vi "run.vi"(8 "error in (no error)":errorcluster, 9 "closeEvent":refnum<user-event>, 10 "snapperEvents":T1, 11 "Views.lvlib:Camera.lvlib:Snapper in":refnum<class "Snapper.lvclass">) -> (0 "error out":errorcluster, 3 "Views.lvlib:Camera.lvlib:Snapper out":refnum<class "Snapper.lvclass">)   [LabVIEW 2009, in "Views.lvlib" / "Camera.lvlib" / "Snapper.lvclass"]
uses:
  Snapper.lvclass
  C:/Program Files/National Instruments/LabVIEW 2009/resource/objmgr/IMAQImage.rc
panel:
  in  "Scrollbar":i32(c297)
  out "Path":path
  out "Boolean":bool=TRUE
  in  "stop":bool
  in  "snap":bool
  out "Image":T2(plugin-control)
  in  "close":bool
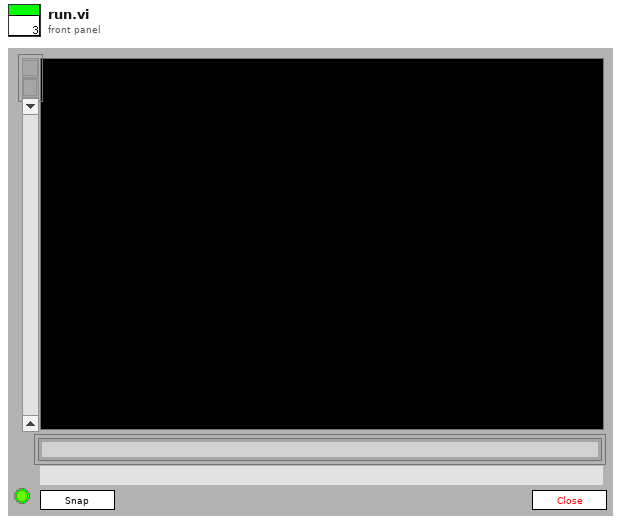
[diagram p1: front panel]
types:
  T1 = cluster{"frontEndEvents":cluster{"snapShotEvent":refnum<user-event>, "stopShooting":refnum<user-event>, "userSnapShot":refnum<user-event>}, "backEndEvents":cluster{"picture":refnum<user-event>}}
  T2 = typedef "IMAQ Image.ctl" = refnum<image>
  T3 = cluster{"snapShotEvent":refnum<user-event>, "stopShooting":refnum<user-event>, "userSnapShot":refnum<user-event>}
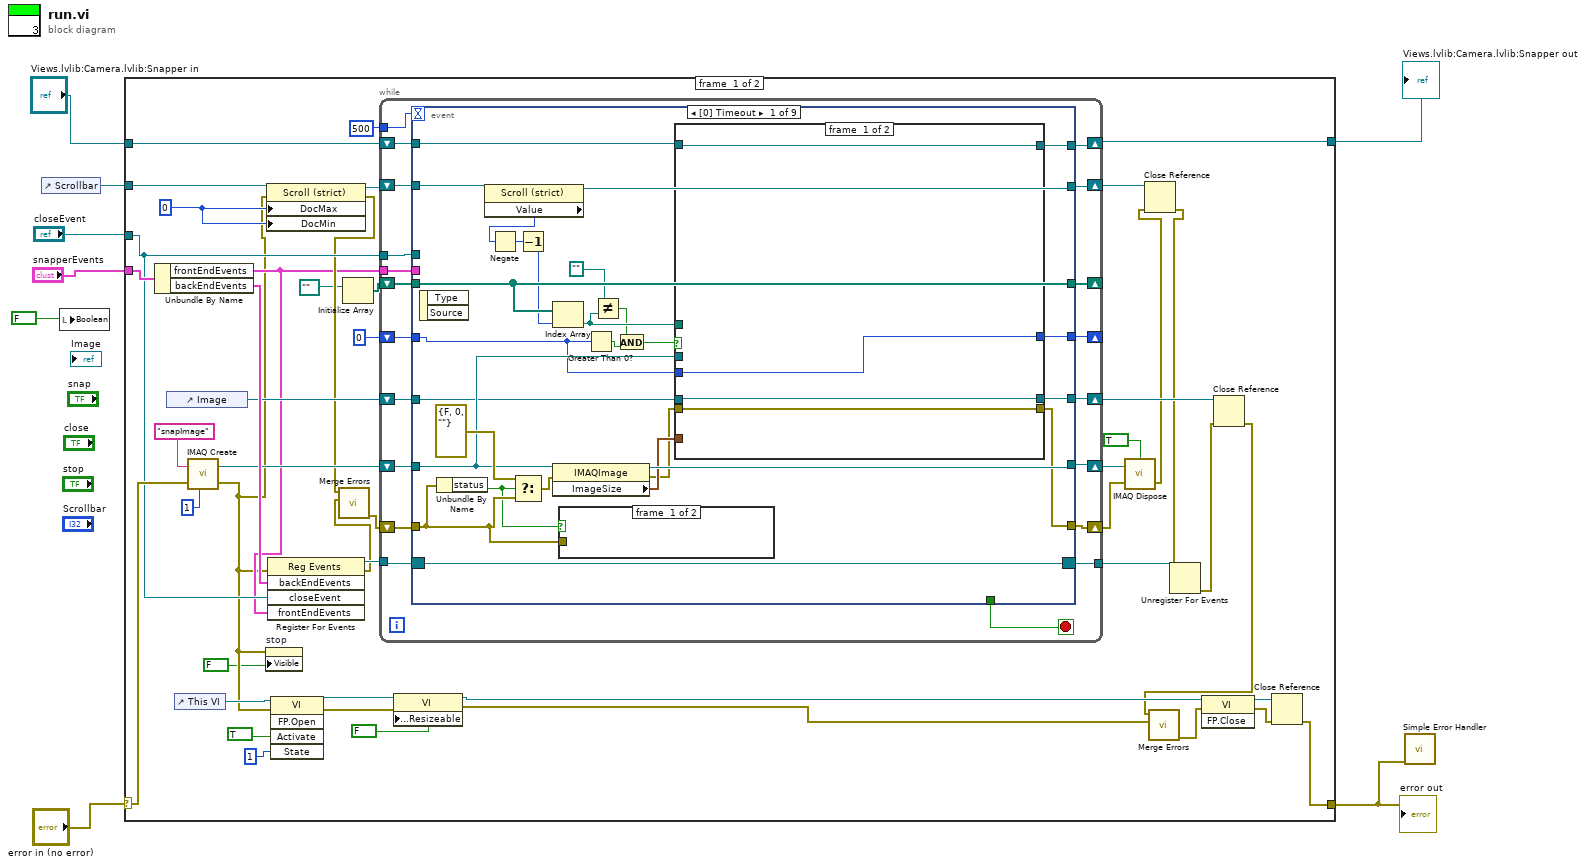
[diagram p0: block diagram]
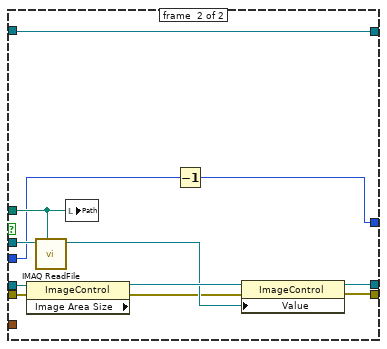
[diagram p2: hidden frame]
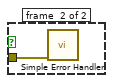
[diagram p3: hidden frame]
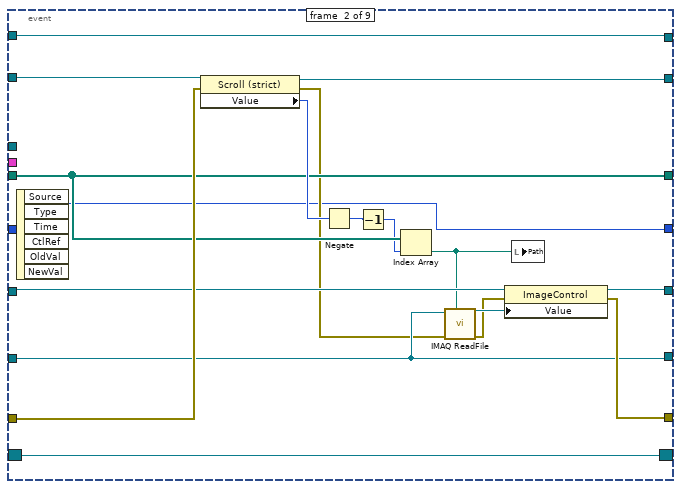
[diagram p4: hidden frame]
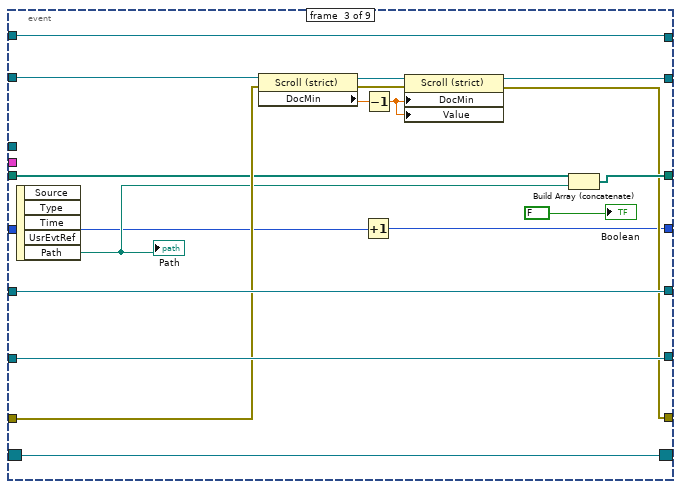
[diagram p5: hidden frame]
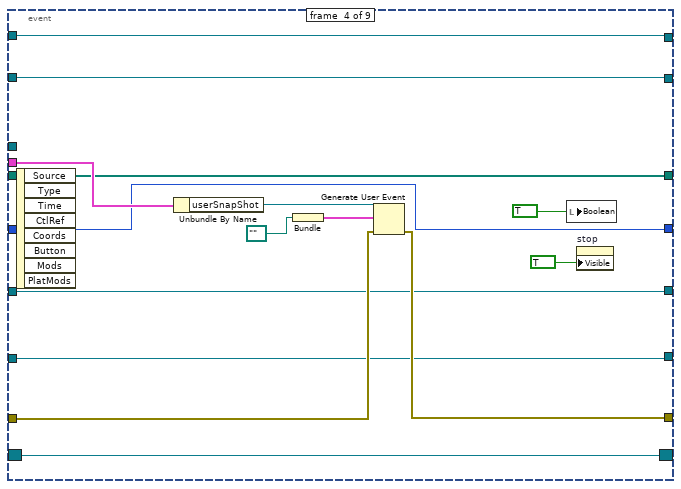
[diagram p6: hidden frame]
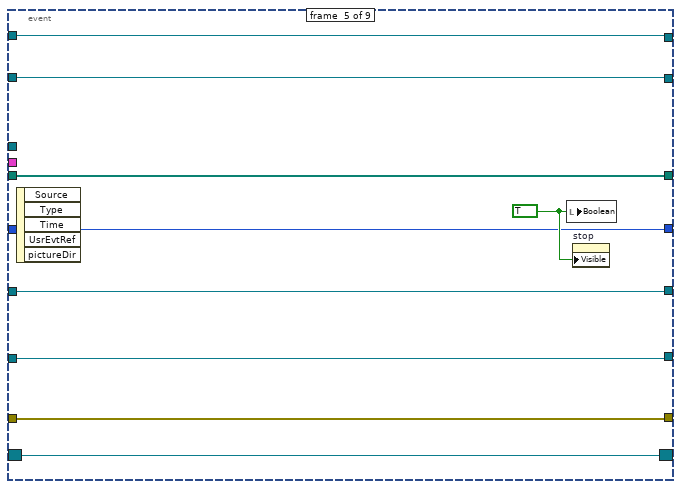
[diagram p7: hidden frame]
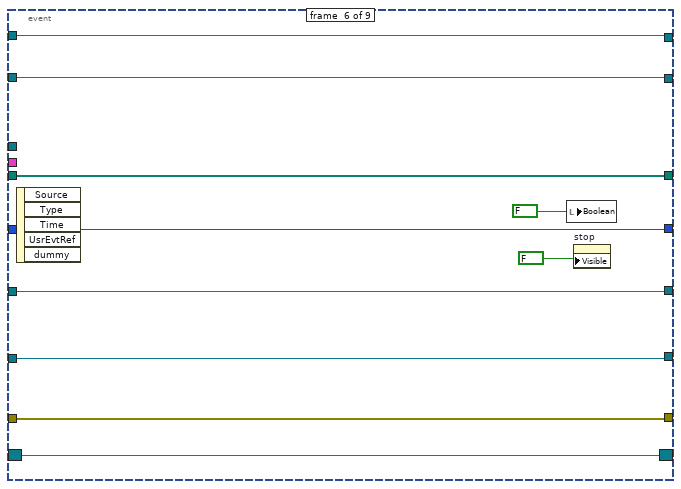
[diagram p8: hidden frame]
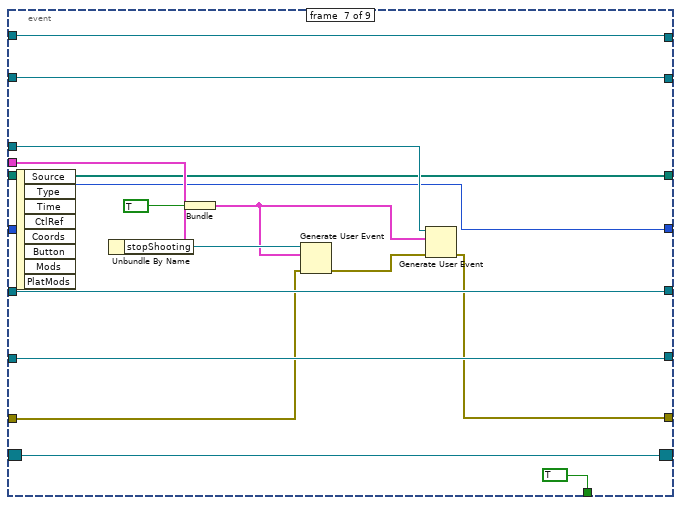
[diagram p9: hidden frame]
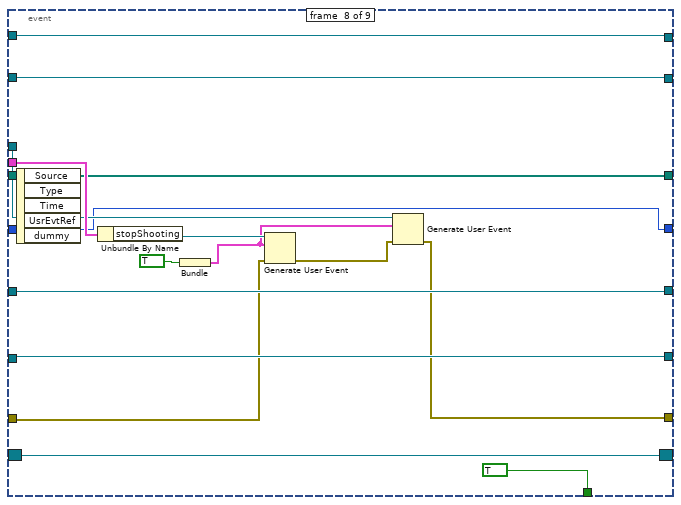
[diagram p10: hidden frame]
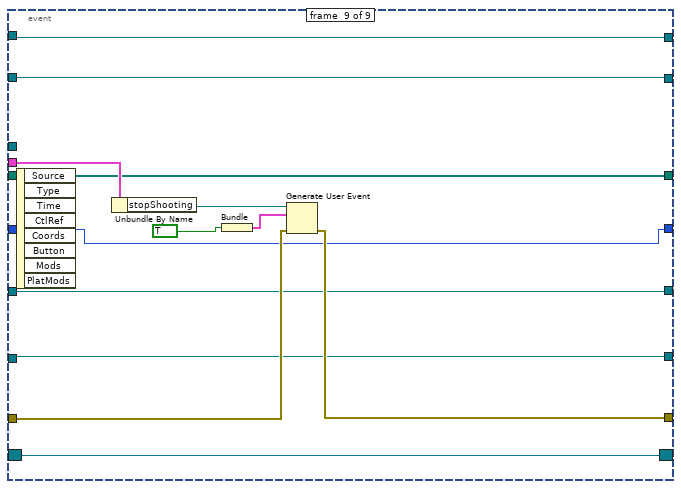
[diagram p11: hidden frame]
diagram:
  n1 = control-ref of="Scrollbar"() -> (w2:refnum<vi>)
  n2 = local write "Boolean"(FALSE) -> ()
  n3 = case shown="No Error" "error in (no error)" {
    selector: "error in (no error)" -> [w48 w235]
    tunnel: [w34 w235] -> w1
    tunnel: [w21 w234] -> w6
    tunnel: "Views.lvlib:Camera.lvlib:Snapper in" -> [w22 w234]
    tunnel: "snapperEvents" -> [w54 _]
    tunnel: "closeEvent" -> [w33 _]
    tunnel: w2 -> [w32 _]
    frame #0 {
      w30 = 0
      n4 = Unbundle By Name(w54) -> ("frontEndEvents"=w16:T3, "backEndEvents"=w52:cluster{"picture":refnum<user-event>})
      n5 = control-ref of="Image"() -> (w47:refnum<vi>)
      n6 = control-ref of="This VI"() -> (w40:refnum<vi>)
      n7 = call "IMAQ Create"("Image Name"="snapImage", "Image Type"=1, "error in (no error)"=w48) -> ("New Image"=w50:T2, "error out"=w15:errorcluster)  [unwired: 2 in]
      n8 = property on="stop" class="Bool (strict)"(error in=w15, "Visible"=FALSE) -> ()  [unwired: 1 in, 2 out]
      n9 = property class="Scroll (strict)"(reference=w32, error in=w15, "DocMax"=w30, "DocMin"=w30) -> (reference out=w31:refnum<vi>, error out=w29:errorcluster)
      n10 = register-events(error in=w15, w52, w33, w16) -> (reference out=w53:refnum<event-registration>, error out=w28:errorcluster)  [unwired: 1 in]
      n11 = invoke class="VI" method="FP.Open"(reference=w40, error in=w15, "Activate"=TRUE, "State"=1) -> (reference out=w36:refnum<vi>, error out=w35:errorcluster)  [unwired: 1 in, 3 out]
      n12 = call <vilib>:"Merge Errors.vi"("error in 2 (no error)"=w28, "error in 1 (no error)"=w29) -> ("error out"=w27:errorcluster)  [unwired: 5 in]
      n13 = Initialize Array(path "") -> (w25:path[])  [unwired: 1 in]
      n14 = while {
        tunnel: w16 -> [w74]
        tunnel: w53 -> [w73]
        shift-right: [w66] -> w45
        shift-left: w50 -> [w71]
        shift-right: [w69] -> w42
        shift-left: w47 -> [w70]
        shift-right: [w68] -> w44
        shift-left: w27 -> [w72]
        tunnel: [w67] -> w43
        tunnel: w33 -> [w64]
        shift-right: [w62] -> w26
        shift-left: w31 -> [w63]
        shift-right: [w61] -> _
        shift-left: w25 -> [w60]
        tunnel: 500 -> [w59]
        shift-right: [w57] -> w21
        shift-left: w22 -> [w58]
        shift-right: [w55] -> _
        shift-left: 0 -> [w56]
        stop <- w65 stop-if-true
        n15 = event shown="[0] Timeout" {
          selector: w73 -> [w101 w130 w154 w164 w178 w188 w203 w219 w227]
          dyn-events: [w101 w130 w154 w164 w178 w188 w203 w219 w227] -> w67
          timeout: w59 -> [_ _ _ _ _ _ _ _ _]
          tunnel: w74 -> [_ _ _ w169 _ _ w197 w216 w233]
          tunnel: w72 -> [w90 w134 w143 w166 w172 w181 w194 w213 w229]
          tunnel: w71 -> [w93 w125 w144 w163 w177 w187 w202 w218 w226]
          tunnel: w70 -> [w82 w133 w145 w162 w176 w186 w201 w217 w225]
          tunnel: [w91 w125 w144 w163 w177 w187 w202 w218 w226] -> w66
          tunnel: [w77 w132 w145 w162 w176 w186 w201 w217 w225] -> w69
          tunnel: [w76 w131 w139 w165 w172 w181 w199 w209 w228] -> w68
          tunnel: [_ _ _ _ _ _ TRUE TRUE _] -> w65
          tunnel: w64 -> [_ _ _ _ _ _ w200 w212 _]
          tunnel: w63 -> [w98 w136 w153 w159 w175 w184 w192 w208 w224]
          tunnel: [w94 w135 w149 w159 w175 w184 w192 w208 w224] -> w62
          tunnel: [w99 w128 w147 w158 w174 w183 w191 w207 w223] -> w61
          tunnel: w60 -> [w99 w128 w142 w158 w174 w183 w191 w207 w223]
          tunnel: w58 -> [w79 w122 w146 w157 w173 w182 w190 w206 w222]
          tunnel: [w78 w122 w146 w157 w173 w182 w190 w206 w222] -> w57
          tunnel: w56 -> [w83 w119 w138 w155 w170 w179 w189 w205 w221]
          tunnel: [w75 w119 w137 w155 w170 w179 w189 w205 w221] -> w55
          event #0 {
            n16 = event-data() -> ()  [unwired: 1 in, 2 out]
            n17 = Unbundle By Name(w90) -> ("status"=w89:bool)
            n18 = property class="Scroll (strict)"(reference=w98) -> (reference out=w94:refnum<vi>, "Value"=w97:i32)  [unwired: 1 in, 1 out]
            n19 = Negate(x=w97) -> (-x=w96:i32)
            n20 = Select(t=errorcluster {"status"=FALSE, "code"=0, "source"=""} ("error out"), s=w89, f=w90) -> (s? t:f=w92:errorcluster)
            n21 = Decrement(x=w96) -> (x-1=w95:i32)
            n22 = Index Array(array=w99, index=w95) -> (element=w87:path)
            n23 = property class="IMAQImage"(reference=w93, error in=w92) -> (reference out=w91:T2, error out=w80:errorcluster, "ImageSize"=w81:cluster{"x":i32, "y":i32})
            n24 = case shown="True" w89 {
              tunnel: w90 -> [_ w118]
              frame #0 {
              }
              frame #1 {
                n25 = call <vilib>:"Simple Error Handler.vi"("error in (no error)"=w118) -> ()  [unwired: 4 in, 5 out]
              }
            }
            n26 = Greater Than 0?(x=w83) -> (x > 0?=w84:bool)
            n27 = Not Equal?(x=path "", y=w87) -> (x != y?=w85:bool)
            n28 = And(x=w85, y=w84) -> (x .and. y?=w86:bool)
            n29 = case shown="True" w86 {
              tunnel: w93 -> [_ w117]
              tunnel: w87 -> [_ w116]
              tunnel: w83 -> [w102 w109]
              tunnel: w82 -> [w105 w115]
              tunnel: w80 -> [w104 w114]
              tunnel: w81 -> [_ _]
              tunnel: w79 -> [w103 w107]
              tunnel: [w103 w107] -> w78
              tunnel: [w105 w111] -> w77
              tunnel: [w104 w110] -> w76
              tunnel: [w102 w108] -> w75
              frame #0 {
              }
              frame #1 {
                n30 = property class="ImageControl" props=["Image Area Size"](reference=w115, error in=w114) -> (reference out=w113:refnum<vi>, error out=w106:errorcluster)  [unwired: 1 out]
                n31 = call "IMAQ ReadFile"("File Path"=w116, "Image"=w117) -> ("Image Out"=w112:T2)  [unwired: 5 in, 4 out]
                n32 = local write "Path"(w116) -> ()
                n33 = Decrement(x=w109) -> (x-1=w108:i32)
                n34 = property class="ImageControl"(reference=w113, error in=w106, "Value"=w112) -> (reference out=w111:refnum<vi>, error out=w110:errorcluster)
              }
            }
          }
          event #1 {
            n35 = event-data() -> ()  [unwired: 1 in, 6 out]
            n36 = property class="Scroll (strict)"(reference=w136, error in=w134) -> (reference out=w135:refnum<vi>, error out=w124:errorcluster, "Value"=w129:i32)
            n37 = Negate(x=w129) -> (-x=w121:i32)
            n38 = Decrement(x=w121) -> (x-1=w120:i32)
            n39 = Index Array(array=w128, index=w120) -> (element=w126:path)
            n40 = call "IMAQ ReadFile"("File Path"=w126, "error in (no error)"=w124, "Image"=w125) -> ("error out"=w123:errorcluster, "Image Out"=w127:T2)  [unwired: 4 in, 3 out]
            n41 = property class="ImageControl"(reference=w133, error in=w123, "Value"=w127) -> (reference out=w132:refnum<vi>, error out=w131:errorcluster)
            n42 = local write "Path"(w126) -> ()
          }
          event #2 {
            n43 = event-data() -> ("Path"=w141:path)  [unwired: 1 in, 4 out]
            "Path" <- w141
            n44 = property class="Scroll (strict)"(reference=w153, error in=w143) -> (reference out=w152:refnum<vi>, error out=w151:errorcluster, "DocMin"=w150:dbl)
            n45 = Increment(x=w138) -> (x+1=w137:i32)
            n46 = Decrement(x=w150) -> (x-1=w140:dbl)
            n47 = property class="Scroll (strict)"(reference=w152, error in=w151, "DocMin"=w140, "Value"=w140) -> (reference out=w149:refnum<vi>, error out=w139:errorcluster)
            n48 = Build Array (concatenate)(w142, w141) -> (w147:path[])
            "Boolean" <- FALSE
          }
          event #3 {
            n49 = event-data() -> ()  [unwired: 1 in, 8 out]
            n50 = Unbundle By Name(w169) -> ("userSnapShot"=w168:refnum<user-event>)
            n51 = Bundle(path "") -> (w167:cluster{path})  [unwired: 1 in]
            n52 = Generate User Event(user event=w168, event data cluster=w167, error in=w166) -> (error out=w165:errorcluster)  [unwired: 1 out]
            n53 = local write "Boolean"(TRUE) -> ()
            n54 = property on="stop" class="Bool (strict)"("Visible"=TRUE) -> ()  [unwired: 2 in, 2 out]
          }
          event #4 {
            w171 = TRUE
            n55 = event-data() -> ()  [unwired: 1 in, 5 out]
            n56 = local write "Boolean"(w171) -> ()
            n57 = property on="stop" class="Bool (strict)"("Visible"=w171) -> ()  [unwired: 2 in, 2 out]
          }
          event #5 {
            n58 = event-data() -> ()  [unwired: 1 in, 5 out]
            n59 = local write "Boolean"(FALSE) -> ()
            n60 = property on="stop" class="Bool (strict)"("Visible"=FALSE) -> ()  [unwired: 2 in, 2 out]
          }
          event #6 {
            n61 = event-data() -> ()  [unwired: 1 in, 8 out]
            n62 = Unbundle By Name(w197) -> ("stopShooting"=w196:refnum<user-event>)
            n63 = Bundle(TRUE) -> (w195:cluster{bool})  [unwired: 1 in]
            n64 = Generate User Event(user event=w196, event data cluster=w195, error in=w194) -> (error out=w193:errorcluster)  [unwired: 1 out]
            n65 = Generate User Event(user event=w200, event data cluster=w195, error in=w193) -> (error out=w199:errorcluster)  [unwired: 1 out]
          }
          event #7 {
            n66 = event-data() -> ()  [unwired: 1 in, 5 out]
            n67 = Unbundle By Name(w216) -> ("stopShooting"=w214:refnum<user-event>)
            n68 = Bundle(TRUE) -> (w210:cluster{bool})  [unwired: 1 in]
            n69 = Generate User Event(user event=w214, event data cluster=w210, error in=w213) -> (error out=w211:errorcluster)  [unwired: 1 out]
            n70 = Generate User Event(user event=w212, event data cluster=w210, error in=w211) -> (error out=w209:errorcluster)  [unwired: 1 out]
          }
          event #8 {
            n71 = event-data() -> ()  [unwired: 1 in, 8 out]
            n72 = Unbundle By Name(w233) -> ("stopShooting"=w232:refnum<user-event>)
            n73 = Bundle(TRUE) -> (w230:cluster{bool})  [unwired: 1 in]
            n74 = Generate User Event(user event=w232, event data cluster=w230, error in=w229) -> (error out=w228:errorcluster)  [unwired: 1 out]
          }
        }
      }
      n75 = property class="VI"(reference=w36, error in=w35, "Front Panel.Resizeable"=FALSE) -> (reference out=w13:refnum<vi>, error out=w10:errorcluster)
      n76 = call "IMAQ Dispose"("All Images? (No)"=TRUE, "Image"=w45, "error in (no error)"=w44) -> ("error out"=w20:errorcluster)  [unwired: 3 in]
      n77 = Close Reference(reference=w26, error in (no error)=w20) -> (error out=w19:errorcluster)
      n78 = Unregister For Events(event registration refnum=w43, error in=w19) -> (error out=w41:errorcluster)
      n79 = Close Reference(reference=w42, error in (no error)=w41) -> (error out=w11:errorcluster)
      n80 = call <vilib>:"Merge Errors.vi"("error in 2 (no error)"=w10, "error in 1 (no error)"=w11) -> ("error out"=w12:errorcluster)  [unwired: 5 in]
      n81 = invoke class="VI" method="FP.Close"(reference=w13, error in=w12) -> (reference out=w18:refnum<vi>, error out=w17:errorcluster)  [unwired: 1 in, 1 out]
      n82 = Close Reference(reference=w18, error in (no error)=w17) -> (error out=w34:errorcluster)
    }
    frame #1 {
    }
  }
  "error out" <- w1
  "Views.lvlib:Camera.lvlib:Snapper out" <- w6
  n83 = call <vilib>:"Simple Error Handler.vi"("error in (no error)"=w1) -> ()  [unwired: 4 in, 5 out]
